vi "garabato PLL-FM.vi"() -> ()   [LabVIEW 2019]
uses:
  <vilib>/Analysis/3filter.llb/Filter Passband Type.ctl
  <vilib>/measure/maspectr.llb/FFT Power Spectrum and PSD for 1 Chan.vi
  <vilib>/Waveform/WDTOps.llb/WDT Get Waveform Time Array DBL.vi
  <vilib>/express/express analysis/Spectral/Block/exnSpectralBlock spectral measurements peak poly.vi
  <vilib>/express/express analysis/Spectral/Block/exnSpectralBlock spectral measurements peak WFM.vi
  <vilib>/Analysis/3filter.llb/Butterworth Filter (DBL).vi
  <vilib>/express/express analysis/Spectral/XNode/ExpressSpectralMeasurementsBlockNode.xnode
  <vilib>/measure/NI_MABase.lvlib
  <vilib>/Analysis/NI_AALPro.lvlib
  <vilib>/measure/NI_MAPro.lvlib
  <vilib>/Analysis/NI_AALBase.lvlib
panel:
  in  "high cutoff freq: fh":dbl=4000.0 format="%#_13g"
  in  "Boolean":bool
  in  "stop":bool
  out "Espectro Recuperado":cluster{"f0":dbl, "df":dbl, "magnitude":dbl[]}(graph)={"f0"=0.0, "df"=0.4778519417475728, "magnitude"=array[46144 elements]}
  out "Señal Recuperada":waveform(dbl)(graph)
  out "dt":dbl=2.2675736961451248e-05
  out "Frecuencia del mensaje":dbl=2363.9020464018645
  in  "Datos del mensaje":T1={"Frecuencia del mensaje"=2363.9020464018645, "Amplitud del mensaje"=1.4353408200619526, "Fase del mensaje"=0.0} {"Fase del mensaje" scale=0.0..90.0; "Amplitud del mensaje" scale=0.0..10.0; "Frecuencia del mensaje" scale=0.0..3500.0}
  in  "?":T2(tab)=enum."Señal modulada en FM"
  out "Mensaje  en frecuencia":cluster{"f0":dbl, "df":dbl, "magnitude":dbl[]}(graph)={"f0"=0.0, "df"=0.4778519417475728, "magnitude"=array[46144 elements]}
  out "Mensaje en tiempo":waveform(dbl)(graph)={"t0"=timestamp(0 s since 1904-01-01), "dt"=2.2675736961451248e-05, "Y"=array[92288 elements]}
  out "Mensaje modulado en frecuencia":cluster{"f0":dbl, "df":dbl, "magnitude":dbl[]}(graph)={"f0"=0.0, "df"=0.4778519417475728, "magnitude"=array[46144 elements]}
  out "Mensaje modulado en tiempo":waveform(dbl)(graph)={"t0"=timestamp(0 s since 1904-01-01), "dt"=2.2675736961451248e-05, "Y"=array[92288 elements]}
  out "Delta w":dbl=1700.0
  out "Beta":sgl=0.06851102
  in  "Kf":dbl=1700.0
  out "Señal Detectada":waveform(dbl)(graph)={"t0"=timestamp(0 s since 1904-01-01), "dt"=2.2675736961451248e-05, "Y"=array[92288 elements]}
  out "Espectro Detectado":cluster{"f0":dbl, "df":dbl, "magnitude":dbl[]}(graph)={"f0"=0.0, "df"=0.4778519417475728, "magnitude"=array[46144 elements]}
  in  "Datos de la portadora":T3={"Frecuencia de la portadora"=24813.527253217217, "Amplitud de la portadora"=5.0000184051088805, "Fase de la portadora"=0.0} {"Fase de la portadora" scale=0.0..90.0; "Amplitud de la portadora" scale=0.0..10.0; "Frecuencia de la portadora" scale=0.0..45000.0}
  in  "Muestreo":cluster{"Fs":dbl, "#s":dbl}={"Fs"=1000000.0, "#s"=1000000.0} {"Fs" format="%.2p"}
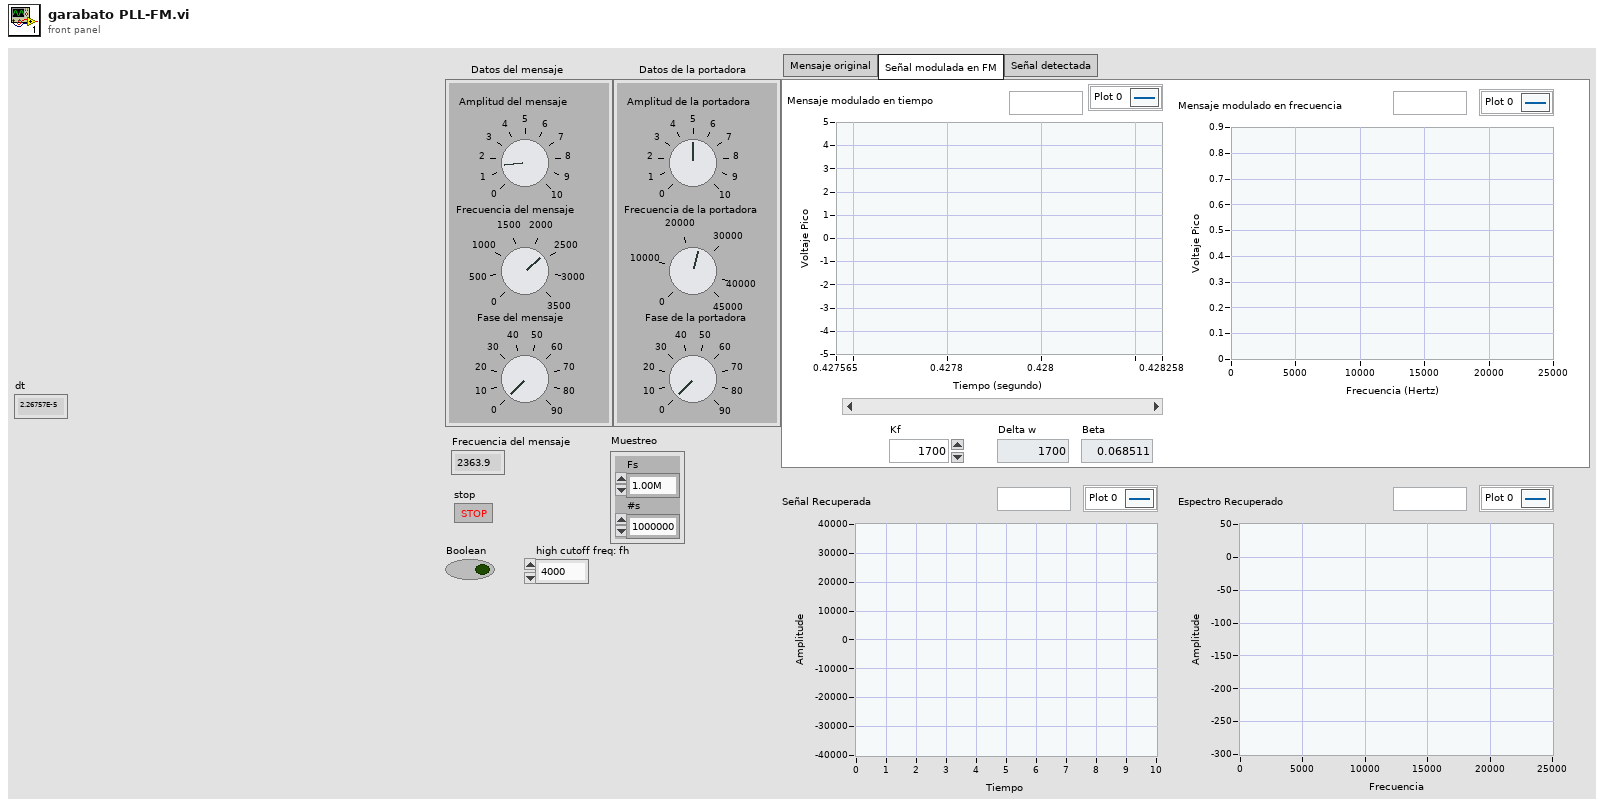
[diagram p1: front panel]
types:
  T1 = cluster{"Frecuencia del mensaje":dbl, "Amplitud del mensaje":dbl, "Fase del mensaje":dbl}
  T2 = enum32{"Mensaje original", "Señal modulada en FM", "Señal detectada"}
  T3 = cluster{"Frecuencia de la portadora":dbl, "Amplitud de la portadora":dbl, "Fase de la portadora":dbl}
  T4 = typedef "NI_AALBase.lvlib/Filter Passband Type.ctl" = enum32{"Lowpass", "Highpass", "Bandpass", "Bandstop"}
  T5 = cluster{"averaging mode":u16, "weighting mode":u16, "number of averages":u32}
  T6 = cluster{"dB On (F)":bool, "unwrap phase (F)":bool, "convert to degree (F)":bool}
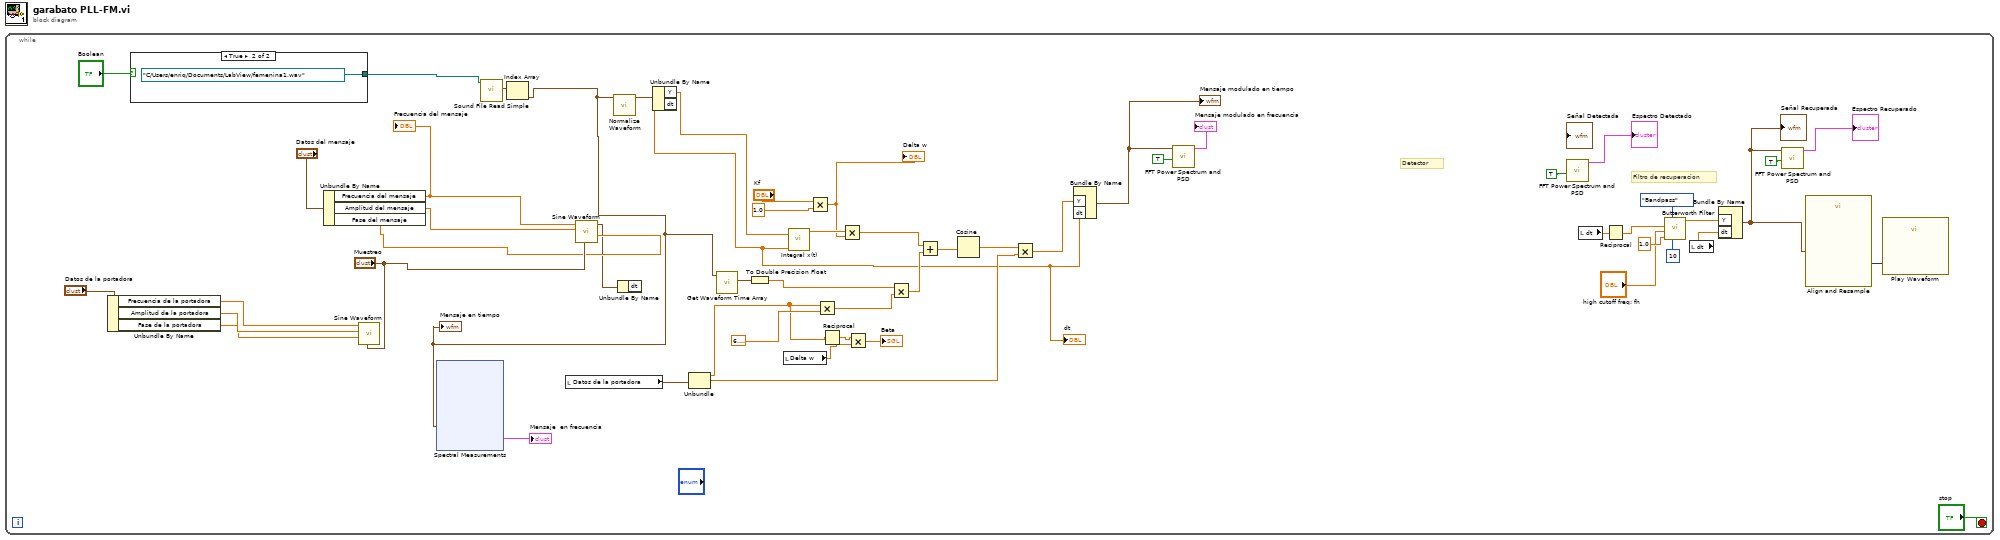
[diagram p0: block diagram]
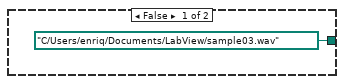
[diagram p2: hidden frame]
diagram:
  n1 = while {
    stop <- "stop" stop-if-true
    # "Filtro de recuperacion"
    # "Detector"
    n2 = Unbundle By Name("Datos de la portadora") -> ("Frecuencia de la portadora"=w54:dbl, "Amplitud de la portadora"=w53:dbl, "Fase de la portadora"=w42:dbl)
    n3 = case shown="True" "Boolean" {
      tunnel: [path "C:/Users/enriq/Documents/LabView/sample03.wav" ("path") path "C:/Users/enriq/Documents/LabView/femenina1.wav" ("path")] -> w13
      frame False {
      }
      frame True {
      }
    }
    n4 = Unbundle By Name("Datos del mensaje") -> ("Frecuencia del mensaje"=w32:dbl, "Amplitud del mensaje"=w31:dbl, "Fase del mensaje"=w30:dbl)
    "Frecuencia del mensaje" <- w32
    n5 = call <vilib>:"Sine Waveform.vi"("sampling info"="Muestreo", "phase"=w42, "amplitude"=w53, "frequency"=w54) -> ()  [unwired: 6 in, 2 out]
    n6 = call <vilib>:"Sound File Read Simple.vi"("path"=w13) -> ("data"=w14:waveform(dbl)[])  [unwired: 7 in, 3 out]
    n7 = Index Array(array=w14) -> (element=w1:waveform(dbl))  [unwired: 1 in]
    "Mensaje en tiempo" <- w1
    n8 = xnode "Spectral Measurements"("Signals"=w1) -> ("FFT - (Peak)"=→"Mensaje  en frecuencia":cluster{"f0":dbl, "df":dbl, "magnitude":dbl[]})  [unwired: 2 in, 3 out]
    n9 = local read "Datos de la portadora"() -> (w50:T3)
    n10 = call <vilib>:"Sine Waveform.vi"("sampling info"="Muestreo", "phase"=w30, "amplitude"=w31, "frequency"=w32) -> ("signal out"=w7:waveform(dbl))  [unwired: 6 in, 1 out]
    n11 = call <vilib>:"Normalize Waveform.vi"("waveform in"=w1) -> ("normalized waveform"=w2:waveform(dbl))  [unwired: 7 in, 3 out]
    n12 = Unbundle By Name(w7) -> ()  [unwired: 1 out]
    n13 = Unbundle By Name(w2) -> ("Y"=w3:dbl[], "dt"=w4:dbl)
    "dt" <- w4
    n14 = Unbundle(w50) -> ("Frecuencia de la portadora"=w16:dbl, "Amplitud de la portadora"=w43:dbl)  [unwired: 1 out]
    n15 = call-poly <vilib>:"Get Waveform Time Array.vi"("waveform in"=w1) -> ("X array"=w51:timestamp[])  [unwired: 9 in, 1 out]
    n16 = To Double Precision Float(number=w51) -> (double precision float=w48:dbl[])
    n17 = local read "Delta w"() -> (w38:dbl)
    n18 = call <vilib>:"Integral x(t).vi"("dt"=w4, "X"=w3) -> ("Integral X"=w55:dbl[])  [unwired: 8 in, 1 out]
    n19 = Multiply(x="Kf", y=1.0) -> (x*y=w37:dbl)
    "Delta w" <- w37
    n20 = Multiply(x=w16, y=6.283185307179586) -> (x*y=w40:dbl)
    n21 = Reciprocal(x=w16) -> (1/x=w39:dbl)
    n22 = Multiply(x=w55, y=w37) -> (x*y=w47:dbl[])
    n23 = Multiply(x=w39, y=w38) -> (x*y=→"Beta":dbl)
    n24 = Multiply(x=w48, y=w40) -> (x*y=w46:dbl[])
    n25 = Add(x=w47, y=w46) -> (x+y=w45:dbl[])
    n26 = Cosine(x=w45) -> (cos(x)=w44:dbl[])
    n27 = Multiply(x=w44, y=w43) -> (x*y=w11:dbl[])
    n28 = Bundle By Name("Y"=w11, "dt"=w4) -> (w10:waveform(dbl))  [unwired: 1 in]
    "Mensaje modulado en tiempo" <- w10
    n29 = call-poly <vilib>:"FFT Power Spectrum and PSD.vi"("dB On (F)"=TRUE, "time signal"=w10) -> ("Power Spectrum / PSD"=→"Mensaje modulado en frecuencia":cluster{"f0":dbl, "df":dbl, "magnitude":dbl[]})  [unwired: 6 in, 3 out]
    n30 = call-poly <vilib>:"FFT Power Spectrum and PSD.vi"("dB On (F)"=TRUE) -> ("Power Spectrum / PSD"=→"Espectro Detectado":cluster{"f0":dbl, "df":dbl, "magnitude":dbl[]})  [unwired: 7 in, 3 out]
    n31 = local read "dt"() -> (w23:dbl)
    n32 = Reciprocal(x=w23) -> (1/x=w27:dbl)
    n33 = call-poly <vilib>:"Butterworth Filter.vi"("order"=10, "filter type"=Filter_Passband_Type."Bandpass", "low cutoff freq: fl"=1.0 ("high cutoff freq: fh"), "high cutoff freq: fh"="high cutoff freq: fh", "sampling freq: fs"=w27) -> ("Filtered X"=w20:dbl[])  [unwired: 3 in, 1 out]
    n34 = local read "dt"() -> (w24:dbl)
    n35 = Bundle By Name("Y"=w20, "dt"=w24) -> (w5:waveform(dbl))  [unwired: 1 in]
    "Señal Recuperada" <- w5
    n36 = call-poly <vilib>:"FFT Power Spectrum and PSD.vi"("dB On (F)"=TRUE, "time signal"=w5) -> ("Power Spectrum / PSD"=→"Espectro Recuperado":cluster{"f0":dbl, "df":dbl, "magnitude":dbl[]})  [unwired: 6 in, 3 out]
    n37 = call "Align and Resample"("Signals"=w5) -> ("Resampled Signals"=w12:dynamicdata)  [unwired: 8 in, 2 out]
    n38 = call "Play Waveform"("Data"=w12) -> ()  [unwired: 18 in, 1 out]
  }
